vi "UHR-Fleezers Control (host) - 12.7b.vi"() -> ()   [LabVIEW 2012] (continued)
    n2530 = Bundle By Name(cluster=w3378, "Set 1"=w3366, "Set 2"=w3365) -> (→"Trap X AI1 (DMA)":T13)
    n2531 = Cluster To Array(cluster=w3387) -> (array=w3384:string[])
    n2532 = Unbundle(w3244) -> (w3245:u32[])  [unwired: 2 out]
    n2533 = Select(t=-1.0, s="Negate Y Axis", f=1.0) -> (s? t:f=w3328:dbl)
    n2534 = for "Trap Position" {
      tunnel: w3392 -> [w3763] mode=indexing
      tunnel: "Trap Pos. Disp. Downsample" -> [w3762]
      tunnel: w3309 -> [w3760]
      tunnel: w3388 -> [w3759]
      tunnel: w3384 -> [w3757] mode=indexing
      tunnel: [w3756] -> w3298 mode=indexing
      tunnel: w3343 -> [w3754] mode=indexing
      tunnel: w3342 -> [w3752]
      tunnel: w3328 -> [w3751]
      n2535 = call "downsample 1D array - double.vi"("Ave N"=w3762, "Array In"=w3763) -> ("Array Out"=w3761:dbl[])  [unwired: 1 out]
      n2536 = Subtract(x=w3761, y=w3754) -> (x-y=w3755:dbl[])
      n2537 = Multiply(x=w3752, y=w3755) -> (x*y=w3753:dbl[])
      n2538 = Multiply(x=w3751, y=w3753) -> (x*y=w3750:dbl[])
      n2539 = Bundle By Name("Y"=w3750, "dt"=w3760, "t0"=w3759) -> (w3758:waveform(dbl))  [unwired: 1 out]
      n2540 = Set Waveform Attribute(5:w3757, 6:"NI_ChannelName" ("name"), 7:w3758) -> (3:w3756:waveform(dbl))  [unwired: 1 in, 2 out]
    }
    n2541 = To Double Precision Float(number=w3245) -> (double precision float=w3451:dbl[])
    n2542 = local read "Display Period (s)"() -> (w3440:dbl)
    n2543 = Increment(x=w3533) -> (x+1=w3534:dbl)
    n2544 = Index Array(array=w3298, index=0) -> (element=w3302:waveform(dbl))
    n2545 = Index Array(array=w3298, index=1) -> (element=w3297:waveform(dbl))
    n2546 = feedback #7(w3534) -> (w3537:dbl)
    n2547 = Select(t=0, s=w3524, f=w3537) -> (s? t:f=w3530:dbl)
    n2548 = Array Size(array=w3451) -> (size(s)=w3536:i32)
    n2549 = Build Array (concatenate)(w3419, w3555) -> (w3421:waveform(dbl)[])
    "All Signals" <- w3421
    n2550 = Add(x=w3536, y=w3530) -> (x+y=w3531:dbl)
    n2551 = Unbundle By Name(w3302) -> ("Y"=w3303:dbl[])
    n2552 = Divide(x="Bead Sep. Int. Time (s)", y=w3440) -> (x/y=w3338:dbl)
    n2553 = Add(x=w3303, y="FB Trap Pos Offset") -> (x+y=w3301:dbl[])
    "T1 x pos data" <- w3301
    n2554 = Greater?(x=w3531, y=w3533) -> (0:w3532:bool)
    n2555 = feedback #8(w3301) -> (w3340:dbl[])
    n2556 = Build Array (concatenate)(w3301, w3340) -> (w3339:dbl[])
    n2557 = Bundle By Name(cluster=w3302, "Y"=w3301) -> (w3300:waveform(dbl))
    n2558 = Select(t=w3530, s=w3532, f=w3531) -> (s? t:f=w3529:dbl)
    n2559 = feedback-in #7(w3529) -> ()
    n2560 = local read "MCL Scanning"() -> (w3527:bool)
    n2561 = Bundle(w3300, w3297) -> (w3296:cluster{waveform(dbl), waveform(dbl)})  [unwired: 1 out]
    n2562 = Split 1D Array(array=w3339, index=w3338) -> (first subarray=w3332:dbl[])  [unwired: 1 out]
    n2563 = feedback-in #8(w3332) -> ()
    n2564 = Not(x=w3532) -> (.not. x?=w3526:bool)
    n2565 = Cluster To Array(cluster=w3296) -> (array=w3272:waveform(dbl)[])
    "Trap Positions" <- w3272
    n2566 = call-poly <vilib>:"Mean.vi"("X"=w3332) -> ("mean"=w3331:dbl)  [unwired: 1 out]
    "Mean T1 Position (nm)" <- w3331
    n2567 = Subtract(x=w3332, y=w3331) -> (x-y=w3337:dbl[])
    n2568 = Square(x=w3337) -> (x^2=w3336:dbl[])
    n2569 = And(x=w3526, y=w3527) -> (x .and. y?=w3528:bool)
    n2570 = call-poly <vilib>:"Mean.vi"("X"=w3336) -> ("mean"=w3335:dbl)  [unwired: 1 out]
    n2571 = Square Root(x=w3335) -> (sqrt(x)=w3334:dbl)
    n2572 = Or(x=w3528, y=w3524) -> (x .or. y?=w3525:bool)
    n2573 = Equal?(x="Tab Control 6", y=T35."High Res Display") -> (x = y?=w3457:bool)
    n2574 = Multiply(x=10.0, y=w3334) -> (x*y=→"Trap 1 Position RMS (A)":dbl)
    n2575 = case "For displaying the high resolution display (no downsampling)" shown="True" w3457 {
      tunnel: w3423 -> [_ w3783]
      frame False {
      }
      frame True {
        n2576 = Index Array(array=w3783, index="High Res. Display") -> (element=w3784:waveform(dbl))
        n2577 = call <vilib>:"Std Deviation and Variance.vi"("X"=w3784) -> ("mean"=w3791:dbl, "standard deviation"=w3796:dbl)  [unwired: 1 in, 1 out]
        "Mean Intensity" <- w3791
        "Sigma" <- w3796
        n2578 = Subtract(x=w3784, y=w3791) -> (x-y=w3790:waveform(dbl))
        n2579 = Select(t=w3790, s="Subtract mean", f=w3784) -> (s? t:f=→"1 Channel":waveform(dbl))
        n2580 = Divide(x=w3796, y=w3791) -> (x/y=→"Sigma/Mean":dbl)
        n2581 = feedback #9(1) -> (w3785:i32)
        n2582 = Greater Or Equal?(x=w3785, y="Slow mean N ave.") -> (x >= y?=w3798:bool)
        n2583 = Increment(x=w3785) -> (x+1=w3800:i32)
        n2584 = Select(t=1, s=w3798, f=w3800) -> (s? t:f=w3787:i32)
        n2585 = feedback-in #9(w3787) -> ()
        n2586 = feedback #10() -> (w3788:waveform(dbl))  [unwired: 1 out]
        n2587 = case shown="Default" w3785 {
          tunnel: [w3803 w3806] -> w3789
          tunnel: w3788 -> [w3805 _]
          tunnel: w3784 -> [w3804 w3806]
          frame Default {
            n2588 = call-poly <vilib>:"Append Waveforms.vi"("waveform B"=w3804, "waveform A"=w3805) -> ("waveform out"=w3803:waveform(dbl))  [unwired: 1 in, 8 out]
          }
          frame 1 {
          }
        }
        n2589 = feedback-in #10(w3789) -> ()
        n2590 = case shown="True" w3798 {
          tunnel: w3789 -> [_ w3802]
          frame False {
          }
          frame True {
            n2591 = call-poly <vilib>:"Mean.vi"("X"=w3802) -> ("mean"=→"Slow mean":dbl)  [unwired: 1 out]
          }
        }
      }
    }
    n2592 = case "For plotting results of scanning MCL (fluorescence and detection laser images)" shown="True" w3525 {
      tunnel: w3524 -> [_ w3910]
      tunnel: w3533 -> [_ _]
      tunnel: w3423 -> [_ w4039]
      tunnel: w3401 -> [_ w3947]
      tunnel: w3244 -> [_ w3917]
      frame False {
      }
      frame True {
        w3927 = u32 0 items=["Horizontal", "Vertical", "Central", "1st Diagonal", "2nd Diagonal"] ("Type of Symmetry")
        w3954 = u32 0 items=["Horizontal", "Vertical", "Central", "1st Diagonal", "2nd Diagonal"] ("Type of Symmetry")
        w3978 = u32 0 items=["Horizontal", "Vertical", "Central", "1st Diagonal", "2nd Diagonal"] ("Type of Symmetry")
        w3981 = u32 0 items=["Horizontal", "Vertical", "Central", "1st Diagonal", "2nd Diagonal"] ("Type of Symmetry")
        w4010 = u32 0 items=["Horizontal", "Vertical", "Central", "1st Diagonal", "2nd Diagonal"] ("Type of Symmetry")
        n2593 = Unbundle(w3917) -> (w3916:u32[], w3914:u32[], w3912:u32[])
        n2594 = To Double Precision Float(number=w3916) -> (double precision float=w3915:dbl[])
        n2595 = To Double Precision Float(number=w3914) -> (double precision float=w3913:dbl[])
        n2596 = To Double Precision Float(number=w3912) -> (double precision float=w3911:dbl[])
        n2597 = Index Array(array=w4039, index=10) -> (element=w4045:waveform(dbl))
        n2598 = Index Array(array=w4039, index=11) -> (element=w4042:waveform(dbl))
        n2599 = local read "Cycles/step (MCL)"() -> (w3995:u64)
        n2600 = Index Array(array=w4039, index="Channel") -> (element=w4041:waveform(dbl))
        n2601 = Unbundle(w3947) -> ("New Image"=w3946:T2, "New Image"=w3945:T2, "New Image"=w3918:T2, "New Image"=w3919:T2, "New Image"=w3920:T2)
        n2602 = local read "Scan steps (MCL)"() -> (w3906:u64)
        n2603 = Unbundle By Name(w4045) -> ("Y"=w3997:dbl[])
        n2604 = Unbundle By Name(w4042) -> ("Y"=w3999:dbl[])
        n2605 = local read "Scan lines (y)"() -> (w3907:u64)
        n2606 = local read "N APD Samp/step"() -> (w3909:dbl)
        n2607 = Unbundle By Name(w4041) -> ("Y"=w4004:dbl[])
        n2608 = call "downsample 1D array - double.vi"("Ave N"=w3995, "Array In"=w3997) -> ("Array Out"=w3996:dbl[])  [unwired: 1 out]
        n2609 = call "downsample 1D array - double.vi"("Ave N"=w3995, "Array In"=w3999) -> ("Array Out"=w3998:dbl[])  [unwired: 1 out]
        n2610 = call "downsample 1D array - double.vi"("Ave N"=w3995, "Array In"=w4004) -> ("Array Out"=w4003:dbl[])  [unwired: 1 out]
        n2611 = Multiply(x=w3906, y=u64 2) -> (x*y=w3908:u64)
        n2612 = feedback #11(w3913) -> (w3972:dbl[])
        n2613 = Build Array (concatenate)(w3972, w3913) -> (w3971:dbl[])
        n2614 = feedback #12(w3911) -> (w3944:dbl[])
        n2615 = Build Array (concatenate)(w3944, w3911) -> (w3905:dbl[])
        n2616 = Select(t=w3913, s=w3910, f=w3971) -> (s? t:f=w3956:dbl[])
        n2617 = feedback-in #11(w3956) -> ()
        n2618 = Select(t=w3911, s=w3910, f=w3905) -> (s? t:f=w3929:dbl[])
        n2619 = feedback-in #12(w3929) -> ()
        n2620 = feedback #13(w3915) -> (w4065:dbl[])
        n2621 = Build Array (concatenate)(w4065, w3915) -> (w4047:dbl[])
        n2622 = Select(t=w3915, s=w3910, f=w4047) -> (s? t:f=w4051:dbl[])
        n2623 = feedback-in #13(w4051) -> ()
        n2624 = feedback #14(w3996) -> (w4053:dbl[])
        n2625 = Build Array (concatenate)(w4053, w3996) -> (w4044:dbl[])
        n2626 = feedback #15(w4003) -> (w4063:dbl[])
        n2627 = Build Array (concatenate)(w4063, w4003) -> (w4062:dbl[])
        n2628 = feedback #16(w3998) -> (w4055:dbl[])
        n2629 = Build Array (concatenate)(w4055, w3998) -> (w4056:dbl[])
        n2630 = Select(t=w3996, s=w3910, f=w4044) -> (s? t:f=w4000:dbl[])
        n2631 = feedback-in #14(w4000) -> ()
        n2632 = Select(t=w4003, s=w3910, f=w4062) -> (s? t:f=w4002:dbl[])
        n2633 = feedback-in #15(w4002) -> ()
        n2634 = Select(t=w3998, s=w3910, f=w4056) -> (s? t:f=w4001:dbl[])
        n2635 = feedback-in #16(w4001) -> ()
        n2636 = call "integrate 1D array interval - double.vi"("Ave N"=w3909, "Array In"=w3956) -> ("Array Out"=w3967:dbl[])  [unwired: 1 out]
        n2637 = call "integrate 1D array interval - double.vi"("Ave N"=w3909, "Array In"=w3929) -> ("Array Out"=w3940:dbl[])  [unwired: 1 out]
        n2638 = call "integrate 1D array interval - double.vi"("Ave N"=w3909, "Array In"=w4051) -> ("Array Out"=w4050:dbl[])  [unwired: 1 out]
        n2639 = Array Size(array=w3967) -> (size(s)=w3968:i32)
        n2640 = Array Size(array=w3940) -> (size(s)=w3941:i32)
        n2641 = Array Size(array=w4050) -> (size(s)=w4052:i32)
        n2642 = Multiply(x=w3907, y=w3908) -> (x*y=w3970:u64)
        n2643 = Multiply(x=w3907, y=w3908) -> (x*y=w3943:u64)
        n2644 = Multiply(x=w3907, y=w3908) -> (x*y=w4060:u64)
        n2645 = Subtract(x=w3970, y=w3968) -> (x-y=w3961:u64)
        n2646 = call-poly <vilib>:"Mean.vi"("X"=w3967) -> ("mean"=w3958:dbl)  [unwired: 1 out]
        n2647 = Subtract(x=w3943, y=w3941) -> (x-y=w3934:u64)
        n2648 = call-poly <vilib>:"Mean.vi"("X"=w3940) -> ("mean"=w3931:dbl)  [unwired: 1 out]
        n2649 = Subtract(x=w4060, y=w4052) -> (x-y=w3994:u64)
        n2650 = call-poly <vilib>:"Mean.vi"("X"=w4050) -> ("mean"=w3991:dbl)  [unwired: 1 out]
        n2651 = call-poly <vilib>:"Mean.vi"("X"=w4000) -> ("mean"=w3984:dbl)  [unwired: 1 out]
        n2652 = call-poly <vilib>:"Mean.vi"("X"=w4002) -> ("mean"=w3989:dbl)  [unwired: 1 out]
        n2653 = call-poly <vilib>:"Mean.vi"("X"=w4001) -> ("mean"=w3987:dbl)  [unwired: 1 out]
        n2654 = Initialize Array(1.0 ("element"), w3961) -> (w3957:dbl[])
        n2655 = Initialize Array(1.0 ("element"), w3934) -> (w3930:dbl[])
        n2656 = Initialize Array(1.0 ("element"), w3994) -> (w3985:dbl[])
        n2657 = Multiply(x=w3957, y=w3958) -> (x*y=w3959:dbl[])
        n2658 = Multiply(x=w3930, y=w3931) -> (x*y=w3932:dbl[])
        n2659 = Multiply(x=w3985, y=w3991) -> (x*y=w3992:dbl[])
        n2660 = Multiply(x=w3985, y=w3987) -> (x*y=w3988:dbl[])
        n2661 = Multiply(x=w3985, y=w3989) -> (x*y=w3990:dbl[])
        n2662 = Multiply(x=w3985, y=w3984) -> (x*y=w3986:dbl[])
        n2663 = Build Array (concatenate)(w3967, w3959) -> (w3969:dbl[])
        n2664 = Build Array (concatenate)(w3940, w3932) -> (w3942:dbl[])
        n2665 = Build Array (concatenate)(w4050, w3992) -> (w4059:dbl[])
        n2666 = Build Array (concatenate)(w4000, w3986) -> (w4054:dbl[])
        n2667 = Build Array (concatenate)(w4002, w3990) -> (w4058:dbl[])
        n2668 = Build Array (concatenate)(w4001, w3988) -> (w4057:dbl[])
        n2669 = Reshape Array(w3969, w3907, w3908) -> (w3965:dbl[][])
        n2670 = Reshape Array(w3942, w3907, w3908) -> (w3938:dbl[][])
        n2671 = Reshape Array(w4059, w3907, w3908) -> (w4037:dbl[][])
        n2672 = Reshape Array(w4054, w3907, w3908) -> (w4020:dbl[][])
        n2673 = Reshape Array(w4058, w3907, w3908) -> (w4012:dbl[][])
        n2674 = Reshape Array(w4057, w3907, w3908) -> (w4027:dbl[][])
        n2675 = Array Subset(array=w3965, index (col)=0 ("index"), length (col)=w3906) -> (w3964:dbl[][])  [unwired: 2 in]
        n2676 = Array Subset(array=w3965, index (col)=w3906) -> (w3962:dbl[][])  [unwired: 3 in]
        n2677 = Array Subset(array=w3938, index (col)=0 ("index"), length (col)=w3906) -> (w3937:dbl[][])  [unwired: 2 in]
        n2678 = Array Subset(array=w3938, index (col)=w3906) -> (w3935:dbl[][])  [unwired: 3 in]
        n2679 = Array Subset(array=w4027, index (col)=0 ("index"), length (col)=w3906) -> (w4032:dbl[][])  [unwired: 2 in]
        n2680 = Array Subset(array=w4027, index (col)=w3906) -> (w4030:dbl[][])  [unwired: 3 in]
        n2681 = Array Subset(array=w4037, index (col)=0 ("index"), length (col)=w3906) -> (w4036:dbl[][])  [unwired: 2 in]
        n2682 = Array Subset(array=w4037, index (col)=w3906) -> (w4034:dbl[][])  [unwired: 3 in]
        n2683 = Array Subset(array=w4012, index (col)=0 ("index"), length (col)=w3906) -> (w4018:dbl[][])  [unwired: 2 in]
        n2684 = Array Subset(array=w4012, index (col)=w3906) -> (w4016:dbl[][])  [unwired: 3 in]
        n2685 = Array Subset(array=w4020, index (col)=0 ("index"), length (col)=w3906) -> (w4025:dbl[][])  [unwired: 2 in]
        n2686 = Array Subset(array=w4020, index (col)=w3906) -> (w4023:dbl[][])  [unwired: 3 in]
        n2687 = for {
          tunnel: w3964 -> [w4069] mode=indexing
          tunnel: [w4068] -> w3963 mode=indexing
          workers-P: _ -> [_]
          n2688 = Reverse 1D Array(array=w4069) -> (reversed array=w4068:dbl[])
        }
        n2689 = for {
          tunnel: w3937 -> [w4067] mode=indexing
          tunnel: [w4066] -> w3936 mode=indexing
          workers-P: _ -> [_]
          n2690 = Reverse 1D Array(array=w4067) -> (reversed array=w4066:dbl[])
        }
        n2691 = for {
          tunnel: w4032 -> [w4075] mode=indexing
          tunnel: [w4074] -> w4031 mode=indexing
          workers-P: _ -> [_]
          n2692 = Reverse 1D Array(array=w4075) -> (reversed array=w4074:dbl[])
        }
        n2693 = for {
          tunnel: w4036 -> [w4077] mode=indexing
          tunnel: [w4076] -> w4035 mode=indexing
          workers-P: _ -> [_]
          n2694 = Reverse 1D Array(array=w4077) -> (reversed array=w4076:dbl[])
        }
        n2695 = for {
          tunnel: w4018 -> [w4071] mode=indexing
          tunnel: [w4070] -> w4017 mode=indexing
          workers-P: _ -> [_]
          n2696 = Reverse 1D Array(array=w4071) -> (reversed array=w4070:dbl[])
        }
        n2697 = for {
          tunnel: w4025 -> [w4073] mode=indexing
          tunnel: [w4072] -> w4024 mode=indexing
          workers-P: _ -> [_]
          n2698 = Reverse 1D Array(array=w4073) -> (reversed array=w4072:dbl[])
        }
        n2699 = Index Array(array=w4037, index (row)=0) -> (element=→"Waveform Graph":dbl[])  [unwired: 1 in]
        n2700 = Add(x=w3963, y=w3962) -> (x+y=w3949:dbl[][])
        n2701 = Add(x=w3936, y=w3935) -> (x+y=w3922:dbl[][])
        n2702 = Add(x=w4031, y=w4030) -> (x+y=w4029:dbl[][])
        n2703 = Add(x=w4035, y=w4034) -> (x+y=w4009:dbl[][])
        n2704 = Add(x=w4017, y=w4016) -> (x+y=w4015:dbl[][])
        n2705 = Add(x=w4024, y=w4023) -> (x+y=w4022:dbl[][])
        n2706 = Divide(x=w4015, y=2) -> (x/y=w4013:dbl[][])
        n2707 = Divide(x=w4029, y=2) -> (x/y=w3974:dbl[][])
        n2708 = To Single Precision Float(number=w4009) -> (single precision float=w4008:sgl[][])
        n2709 = To Single Precision Float(number=w3949) -> (single precision float=w3953:sgl[][])
        n2710 = To Single Precision Float(number=w3922) -> (single precision float=w3926:sgl[][])
        n2711 = Divide(x=w4022, y=2) -> (x/y=w3976:dbl[][])
        n2712 = Transpose 2D Array(2D array=w4013) -> (transposed array=→"Data map":dbl[][])
        n2713 = To Single Precision Float(number=w3974) -> (single precision float=w3980:sgl[][])
        n2714 = To Single Precision Float(number=w3976) -> (single precision float=w3977:sgl[][])
        n2715 = call "IMAQ ArrayToImage"("Image Pixels (Float)"=w4008, "Image"=w3946) -> ("Image Out"=w4011:T2)  [unwired: 8 in, 1 out]
        n2716 = call "IMAQ ArrayToImage"("Image Pixels (Float)"=w3953, "Image"=w3945) -> ("Image Out"=w3955:T2)  [unwired: 8 in, 1 out]
        n2717 = call "IMAQ ArrayToImage"("Image Pixels (Float)"=w3926, "Image"=w3918) -> ("Image Out"=w3928:T2)  [unwired: 8 in, 1 out]
        n2718 = call "IMAQ ArrayToImage"("Image Pixels (Float)"=w3980, "Image"=w3919) -> ("Image Out"=w3982:T2)  [unwired: 8 in, 1 out]
        n2719 = call "IMAQ Symmetry"("Type of Symmetry"=w4010, "Image Src"=w4011) -> ("Image Dst Out"=w4006:T2)  [unwired: 3 in, 1 out]
        n2720 = call "IMAQ ArrayToImage"("Image Pixels (Float)"=w3977, "Image"=w3920) -> ("Image Out"=w3979:T2)  [unwired: 8 in, 1 out]
        n2721 = call "IMAQ Symmetry"("Type of Symmetry"=w3954, "Image Src"=w3955) -> ("Image Dst Out"=w3951:T2)  [unwired: 3 in, 1 out]
        n2722 = call "IMAQ Symmetry"("Type of Symmetry"=w3927, "Image Src"=w3928) -> ("Image Dst Out"=w3924:T2)  [unwired: 3 in, 1 out]
        n2723 = call "IMAQ Symmetry"("Type of Symmetry"=w3981, "Image Src"=w3982) -> ("Image Dst Out"=→"Detection Laser X":T2)  [unwired: 3 in, 1 out]
        n2724 = call "IMAQ Symmetry"("Type of Symmetry"=w3978, "Image Src"=w3979) -> ("Image Dst Out"=→"Detection Laser Y":T2)  [unwired: 3 in, 1 out]
        n2725 = call "IMAQ Set Simple Calibration"("Calibration Axis Info"=T36 {"Origin Pixel"={"X"=0.0, "Y"=0.0}, "Angle Relative to Horizontal (deg)"=0.0, "Axis Reference"=0}, "Grid Descriptor"=T37 {"X Step"=0.3, "Y Step"=0.3, "Unit"=enum."Undefined"}, "Image"=w4006) -> ("Calibrated Image"=→"APD 1":T2)  [unwired: 7 in, 1 out]
        n2726 = call "IMAQ Set Simple Calibration"("Calibration Axis Info"=T36 {"Origin Pixel"={"X"=0.0, "Y"=0.0}, "Angle Relative to Horizontal (deg)"=0.0, "Axis Reference"=0}, "Grid Descriptor"=T37 {"X Step"=0.3, "Y Step"=0.3, "Unit"=enum."Undefined"}, "Image"=w3951) -> ("Calibrated Image"=→"APD 2":T2)  [unwired: 7 in, 1 out]
        n2727 = call "IMAQ Set Simple Calibration"("Calibration Axis Info"=T36 {"Origin Pixel"={"X"=0.0, "Y"=0.0}, "Angle Relative to Horizontal (deg)"=0.0, "Axis Reference"=0}, "Grid Descriptor"=T37 {"X Step"=0.3, "Y Step"=0.3, "Unit"=enum."Undefined"}, "Image"=w3924) -> ("Calibrated Image"=→"APD 3":T2)  [unwired: 7 in, 1 out]
      }
    }
    n2728 = case "For computing FFTs for display" shown="True" "Compute FFT" {
      tunnel: w3423 -> [_ w4549]
      frame False {
      }
      frame True {
        n2729 = Build Array("FFT 1 Choice 1", "FFT 1 Choice 2", "FFT 2 Choice 1", "FFT 2 Choice 2") -> (w4542:u16[])
        n2730 = Array Size(array=w4549) -> (size(s)=w4548:i32)
        n2731 = feedback-in #17(w4542) -> ()
        n2732 = feedback #17(u16[] [100, 100, 100, 100]) -> (w4543:u16[])
        n2733 = feedback-in #18("# Spectra to Ave.") -> ()
        n2734 = feedback #18("# Spectra to Ave.") -> (w4540:dbl)
        n2735 = Not Equal?(x="# Spectra to Ave.", y=w4540) -> (x != y?=w4539:bool)
        n2736 = Not Equal?(x=w4542, y=w4543) -> (x != y?=w4541:bool)
        n2737 = feedback #19(1.0) -> (w4526:dbl)
        n2738 = Compound Arithmetic op=OR("Reset FFT", w4541, w4539) -> (w4524:bool)
        n2739 = Select(t=1.0, s=w4524, f=w4526) -> (s? t:f=w4528:dbl)
        n2740 = Greater?(x=w4528, y="# Spectra to Ave.") -> (0:w4547:bool)
        n2741 = Increment(x=w4528) -> (x+1=w4527:dbl)
        n2742 = feedback-in #19(w4527) -> ()
        n2743 = local read "DMA Update Period (s)"() -> (w4522:dbl)
        n2744 = Multiply(x="# Spectra to Ave.", y=w4522) -> (x*y=→"Ave. Time (s)":dbl)
        n2745 = Build Array(cluster{"f0":dbl, "df":dbl, "magnitude":dbl[]} {"f0"=0.0, "df"=0.0, "magnitude"=[]} ("PSD")) -> (w4531:cluster{"f0":dbl, "df":dbl, "magnitude":dbl[]}[])
        n2746 = Build Array(w4531, w4531, w4531, w4531) -> (w4533:T46)
        n2747 = feedback #20(w4533) -> (w4538:T46)
        n2748 = for {
          N: 4 -> [_]
          tunnel: w4542 -> [w4571] mode=indexing
          tunnel: w4549 -> [w4572]
          tunnel: w4548 -> [w4574]
          tunnel: w4524 -> [w4567]
          tunnel: w4547 -> [w4566]
          tunnel: "# Spectra to Ave." -> [w4565]
          tunnel: [w4564] -> w4537 mode=indexing
          tunnel: w4538 -> [w4569] mode=indexing
          tunnel: [w4568] -> w4525 mode=indexing
          tunnel: w4528 -> [w4563]
          n2749 = Less?(x=w4571, y=w4574) -> (x < y?=w4573:bool)
          n2750 = Index Array(array=w4572, index=w4571) -> (element=w4570:waveform(dbl))
          n2751 = case shown="True" w4573 {
            tunnel: w4570 -> [_ w4591]
            tunnel: w4569 -> [w4576 w4589]
            tunnel: [w4576 w4577] -> w4568
            tunnel: w4567 -> [_ w4588]
            tunnel: w4566 -> [_ w4581]
            tunnel: w4565 -> [_ w4580]
            tunnel: [cluster{"f0":dbl, "df":dbl, "magnitude":dbl[]} {"f0"=0.0, "df"=0.0, "magnitude"=[]} ("PSD") w4582] -> w4564
            tunnel: w4563 -> [_ w4579]
            frame False {
            }
            frame True {
              n2752 = call <vilib>:"Std Deviation and Variance.vi"("X"=w4591) -> ("mean"=w4592:dbl)  [unwired: 1 in, 2 out]
              n2753 = Subtract(x=w4591, y=w4592) -> (x-y=w4590:waveform(dbl))
              n2754 = xnode "Spectral Measurements"("Signals"=w4590) -> ("PSD"=w4584:cluster{"f0":dbl, "df":dbl, "magnitude":dbl[]})  [unwired: 1 in, 1 out]
              n2755 = case shown="False" w4588 {
                tunnel: w4589 -> [w4601 _]
                tunnel: [w4597 w4606] -> w4577
                tunnel: w4584 -> [w4600 w4607]
                tunnel: w4581 -> [w4599 _]
                frame False {
                  n2756 = Build Array (concatenate)(w4601, w4600) -> (w4598:cluster{"f0":dbl, "df":dbl, "magnitude":dbl[]}[])
                  n2757 = case shown="True" w4599 {
                    tunnel: w4598 -> [w4602 w4605]
                    tunnel: [w4602 w4603] -> w4597
                    frame False {
                    }
                    frame True {
                      n2758 = Delete From Array(array=w4605, index=0) -> (array with subset deleted=w4603:cluster{"f0":dbl, "df":dbl, "magnitude":dbl[]}[])  [unwired: 1 in, 1 out]
                    }
                  }
                }
                frame True {
                  n2759 = Build Array(w4607) -> (w4606:cluster{"f0":dbl, "df":dbl, "magnitude":dbl[]}[])
                }
              }
              n2760 = for {
                tunnel: w4577 -> [w4596] mode=indexing
                tunnel: [w4595] -> w4587 mode=indexing
                workers-P: _ -> [_]
                n2761 = Unbundle By Name(w4596) -> ("magnitude"=w4595:dbl[])
              }
              n2762 = Transpose 2D Array(2D array=w4587) -> (transposed array=w4586:dbl[][])
              n2763 = for {
                tunnel: w4586 -> [w4594] mode=indexing
                tunnel: [w4593] -> w4585 mode=indexing
                workers-P: _ -> [_]
                n2764 = Add Array Elements(numeric array=w4594) -> (sum=w4593:dbl)
              }
              n2765 = Select(t=w4580, s=w4581, f=w4579) -> (s? t:f=w4578:dbl)
              n2766 = Divide(x=w4585, y=w4578) -> (x/y=w4583:dbl[])
              n2767 = Bundle By Name(cluster=w4584, "magnitude"=w4583) -> (w4582:cluster{"f0":dbl, "df":dbl, "magnitude":dbl[]})
            }
          }
        }
        n2768 = case shown="True" w4524 {
          tunnel: w4525 -> [w4556 w4562]
          tunnel: [w4556 w4557] -> w4523
          frame False {
          }
          frame True {
            n2769 = Array Subset(array=w4562, index (row)=0 ("index"), length (row)=4 ("length"), index (col)=0 ("index"), length (col)=1 ("length")) -> (w4557:T46)
          }
        }
        n2770 = feedback-in #20(w4523) -> ()
        n2771 = Split 1D Array(array=w4537, index=2) -> (first subarray=→"FFT 1":cluster{"f0":dbl, "df":dbl, "magnitude":dbl[]}[], second subarray=→"FFT 2":cluster{"f0":dbl, "df":dbl, "magnitude":dbl[]}[])
      }
    }
    n2772 = Index Array(array=w3421, index=4) -> (element=w3477:waveform(dbl))
    n2773 = Index Array(array=w3421, index=7) -> (element=w3474:waveform(dbl))
    n2774 = Divide(x="T1 offset_x (mV)", y=1000.0) -> (x/y=w3478:dbl)
    n2775 = feedback-in #21("Calibration") -> ()
    n2776 = feedback #21(u16 1 ("Calibration")) -> (w3496:u16)
    n2777 = Divide(x="T2 offset_x (mV)", y=1000.0) -> (x/y=w3476:dbl)
    n2778 = case shown="2" "Calibration" {
      tunnel: "T1 alpha_x (nm/V)" -> [_ w3870 w3891]
      tunnel: "T1 kappa_x (pN/nm)" -> [_ _ w3881]
      tunnel: "T2 alpha_x (nm/V)" -> [_ w3869 w3889]
      tunnel: "T2 kappa_x (pN/nm)" -> [_ _ w3882]
      tunnel: w3477 -> [w3852 w3867 w3887]
      tunnel: w3474 -> [w3851 w3865 w3885]
      tunnel: [w3852 w3864 w3884] -> w3505
      tunnel: [w3851 w3863 w3883] -> w3504
      tunnel: ["T1 X (V)" ("Label.Text") "T1 X (nm)" ("Label.Text") "T1 X (pN)" ("Label.Text")] -> w3493
      tunnel: ["T2 X (V)" ("Label.Text") "T2 X (nm)" ("Label.Text") "T2 X (pN)" ("Label.Text")] -> w3492
      tunnel: ["Position (V)" ("Label.Text") "Position (nm)" ("Label.Text") "Force (pN)" ("Label.Text")] -> w3494
      tunnel: w3476 -> [_ w3855 w3874]
      tunnel: w3478 -> [_ w3858 w3876]
      tunnel: ["Mean (V)" ("Label.Text") "Mean (nm)" ("Label.Text") "Mean (pN)" ("Label.Text")] -> w3489
      tunnel: ["Difference (V)" ("Label.Text") "Difference (nm)" ("Label.Text") "Difference (pN)" ("Label.Text")] -> w3429
      frame 0, Default {
      }
      frame 1 {
        n2779 = Unbundle By Name(w3867) -> ("Y"=w3871:dbl[])
        n2780 = Unbundle By Name(w3865) -> ("Y"=w3856:dbl[])
        n2781 = Subtract(x=w3871, y=w3858) -> (x-y=w3859:dbl[])
        n2782 = Subtract(x=w3856, y=w3855) -> (x-y=w3857:dbl[])
        n2783 = Multiply(x=w3857, y=w3869) -> (x*y=w3866:dbl[])
        n2784 = Multiply(x=w3870, y=w3859) -> (x*y=w3868:dbl[])
        n2785 = Bundle By Name(cluster=w3865, "Y"=w3866) -> (w3863:waveform(dbl))
        n2786 = Bundle By Name(cluster=w3867, "Y"=w3868) -> (w3864:waveform(dbl))
      }
      frame 2 {
        n2787 = Unbundle By Name(w3887) -> ("Y"=w3892:dbl[])
        n2788 = Unbundle By Name(w3885) -> ("Y"=w3890:dbl[])
        n2789 = Subtract(x=w3890, y=w3874) -> (x-y=w3875:dbl[])
        n2790 = Subtract(x=w3892, y=w3876) -> (x-y=w3877:dbl[])
        n2791 = Compound Arithmetic op=MULTIPLY(w3875, w3889, w3882) -> (w3886:dbl[])
        n2792 = Compound Arithmetic op=MULTIPLY(w3881, w3891, w3877) -> (w3888:dbl[])
        n2793 = Bundle By Name(cluster=w3885, "Y"=w3886) -> (w3883:waveform(dbl))
        n2794 = Bundle By Name(cluster=w3887, "Y"=w3888) -> (w3884:waveform(dbl))
      }
    }
    n2795 = case shown="True" "Read Lateness and Rel Phase" {
      tunnel: w3295 -> [w3807 w3840]
      tunnel: w3294 -> [w3808 w3839]
      tunnel: [w3807 w3812] -> w3471
      tunnel: [w3808 w3811] -> w3470
      frame False {
      }
      frame True {
        n2796 = xnode "Read/Write Control"("FPGA VI Reference In"=w3840, "error in"=w3839) -> ("FPGA VI Reference Out"=w3814:T20, "error out"=w3813:errorcluster, "GI Relative phase"=→"GI relative phase":i16, "Relative phase"=→"Relative phase (AI1)":i16, "AI Late Counter"=→"Late Counter (AI1)":u8, "GI Late Counter"=→"GI Late Counter":u8, "MCL Late Counter"=→"MCL Late Counter":u8, "MCL Relative Phase"=→"Relative Phase (MCL)":i16, "APD Acq Relative Phase"=→"APD Acq Relative Phase":i16, "APD 1 Gate Relative Phase"=→"APD 1 Gate Relative Phase":i16, "APD 2 Gate Relative Phase"=→"APD 2 Gate Relative Phase":i16, "APD Acq Late Counter"=→"APD Acq Late Counter":u8, "APD 1 Gate Late Counter"=→"APD 1 Gate Late Counter":u8, "APD 2 Gate Late Counter"=→"APD 2 Gate Late Counter":u8, "Green FB Relative Phase"=→"Relative phase (Green FB)":i16, "GI Relative phase 2"=→"GI relative phase 2":i16, "GI Late Counter 2"=→"GI Late Counter 2":u8, "Trap Pos FIFO Timeout"=→"Trap Pos FIFO Timeout":u16, "Trap AI FIFO Timeout"=→"Trap AI FIFO Timeout":u16, "RI Late Counter"=→"RI Late Counter":u8, "RI Relative phase"=→"RI relative phase":i16, "Green Late Counter"=→"Green AI Late Counter":u8, "BI Late Counter (AO)"=→"Late Counter (BI AO)":u8, "Blue Late Counter (D)"=→"Late Counter (BI DO)":u8, "BI Relative phase (AO)"=→"Relative phase (BI AO)":i16, "BI Relative phase (D)"=→"Relative phase (BI DO)":i16)
        n2797 = xnode "Read/Write Control"("FPGA VI Reference In"=w3814, "error in"=w3813) -> ("FPGA VI Reference Out"=w3812:T20, "error out"=w3811:errorcluster, "APD 3 Gate Late Counter"=→"APD 3 Gate Late Counter":u8, "APD 3 Gate Relative Phase"=→"APD 3 Gate Relative Phase":i16)
      }
    }
    n2798 = Not Equal?(x=w3496, y="Calibration") -> (x != y?=w3455:bool)
    n2799 = case shown="True" w3455 {
      tunnel: w3494 -> [_ w3845]
      tunnel: w3493 -> [_ w3844]
      tunnel: w3492 -> [_ w3843]
      tunnel: w3489 -> [_ w3842]
      tunnel: w3429 -> [_ w3841]
      frame False {
      }
      frame True {
        n2800 = property on="Force" class="WFChart (strict)"("YScale.NameLbl.Text"=w3845) -> ()  [unwired: 2 in, 2 out]
        n2801 = property on="T2 X" class="DigNum (strict)"("Caption.Text"=w3843) -> ()  [unwired: 2 in, 2 out]
        n2802 = property on="T1 X" class="DigNum (strict)"("Caption.Text"=w3844) -> ()  [unwired: 2 in, 2 out]
        n2803 = property on="Mean" class="DigNum (strict)"("Caption.Text"=w3842) -> ()  [unwired: 2 in, 2 out]
        n2804 = property on="Difference" class="DigNum (strict)"("Caption.Text"=w3841) -> ()  [unwired: 2 in, 2 out]
      }
    }
    n2805 = Unbundle By Name(w3477) -> ("Y"=w3480:dbl[])
    n2806 = Unbundle By Name(w3474) -> ("Y"=w3483:dbl[])
    n2807 = Subtract(x=w3480, y=w3478) -> (x-y=w3481:dbl[])
    n2808 = Subtract(x=w3483, y=w3476) -> (x-y=w3482:dbl[])
    n2809 = Multiply(x=w3482, y="T2 alpha_x (nm/V)") -> (x*y=w3277:dbl[])
    n2810 = Multiply(x="T1 alpha_x (nm/V)", y=w3481) -> (x*y=w3278:dbl[])
    n2811 = Not(x="Trap Trig. Fl.") -> (.not. x?=w3314:bool)
    n2812 = Multiply(x=w3504, y=-1.0) -> (x*y=w3485:waveform(dbl))
    n2813 = Subtract(x=w3278, y=w3277) -> (x-y=w3473:dbl[])
    n2814 = Unbundle By Name(w3504) -> ("Y"=w3445:dbl[])
    n2815 = Unbundle By Name(w3505) -> ("Y"=w3279:dbl[])
    n2816 = Negate(x=w3473) -> (-x=w3275:dbl[])
    n2817 = Build Array(w3505, w3485) -> (→"Force":waveform(dbl)[])
    n2818 = Subtract(x=w3275, y="Offset (nm)") -> (x-y=w3443:dbl[])
    n2819 = call-poly <vilib>:"Mean.vi"("X"=w3445) -> ("mean"=w3281:dbl)  [unwired: 1 out]
    "T2 X" <- w3281
    n2820 = Negate(x=w3445) -> (-x=w3446:dbl[])
    n2821 = call-poly <vilib>:"Mean.vi"("X"=w3279) -> ("mean"=w3282:dbl)  [unwired: 1 out]
    "T1 X" <- w3282
    n2822 = Negate(x=w3281) -> (-x=w3280:dbl)
    n2823 = Bundle By Name(cluster=w3477, "Y"=w3443) -> (w3420:waveform(dbl))
    "Bead Separation" <- w3420
    n2824 = Add(x=w3279, y=w3446) -> (x+y=w3447:dbl[])
    n2825 = Add(x=w3282, y=w3280) -> (x+y=w3491:dbl)
    n2826 = Subtract(x=w3282, y=w3280) -> (x-y=→"Difference":dbl)
    n2827 = Divide(x=w3447, y=2.0) -> (x/y=→"Vec Mean of T1 T2":dbl[])
    n2828 = Divide(x=w3491, y=2.0) -> (x/y=w3449:dbl)
    "Mean" <- w3449
    n2829 = feedback-in #22("Trap Trig. Fl.") -> ()
    n2830 = feedback #22("Trap Trig. Fl.") -> (w3312:bool)
    n2831 = And(x=w3314, y=w3312) -> (x .and. y?=w3313:bool)
    n2832 = case "If have just turned off triggering" shown="True" w3313 {
      tunnel: w3295 -> [_ w3642]
      tunnel: w3294 -> [_ w3641]
      frame False {
      }
      frame True {
        w3640 = FALSE ("FPGA Trap Trig")
        n2833 = xnode "Read/Write Control"("FPGA VI Reference In"=w3642, "error in"=w3641, "FPGA Trap Trig"=w3640) -> ("FPGA VI Reference Out"=w3639:T20, "error out"=w3638:errorcluster)
        n2834 = xnode "Read/Write Control"("FPGA VI Reference In"=w3639, "error in"=w3638, "TTrig?"=w3640) -> ()  [unwired: 2 out]
        n2835 = local write "Initializing"(FALSE ("Initializing")) -> ()
        n2836 = local write "Triggered"(FALSE ("Triggered")) -> ()
        n2837 = local write "Waiting"(FALSE ("Waiting")) -> ()
      }
    }
    n2838 = Not(x=w3312) -> (.not. x?=w3325:bool)
    n2839 = And(x="Trap Trig. Fl.", y=w3325) -> (x .and. y?=w3322:bool)
    n2840 = local read "Tether"() -> (w3450:bool)
    n2841 = Or(x=w3322, y="Reinitialize") -> (x .or. y?=w3308:bool)
    n2842 = feedback #23(w3318) -> (w3323:string)
    n2843 = Select(t=w3318, s=w3322, f=w3323) -> (s? t:f=w3317:string)
    n2844 = Select(t=w3318, s="Reinitialize", f=w3317) -> (s? t:f=w3316:string)
    n2845 = feedback #24(0) -> (w3320:i32)
    n2846 = feedback #25(w3443) -> (w3442:dbl[])
    n2847 = Build Array (concatenate)(w3443, w3442) -> (w3276:dbl[])
    n2848 = case "For determining if there is a tether still" shown="True" w3450 {
      tunnel: w3449 -> [_ w3766]
      frame False {
      }
      frame True {
        n2849 = Greater?(x="Lost Tether Alarm Threshold (pN)", y=w3766) -> (0:w3764:bool)
        n2850 = case shown="True" w3764 {
          frame False {
          }
          frame True {
            w3767 = FALSE ("Value (Signaling)")
            n2851 = flat-sequence {
              frame #0 {
                # "stop only if saving"
                n2852 = local read "Saving..."() -> (w3779:bool)
                n2853 = And(x=w3779, y="TA Cancel Save?") -> (x .and. y?=w3778:bool)
                n2854 = local write "Stop Saving"(w3778) -> ()
              }
              frame #1 {
                n2855 = case shown="True" "TA Green Off?" {
                  frame False {
                  }
                  frame True {
                    w3782 = FALSE ("Fl. Triggered...")
                    n2856 = local write "Fl. Triggered..."(w3782) -> ()
                    n2857 = property on="Green Laser ON" class="Bool (strict)"("Val(Sgnl)"=w3782) -> ()  [unwired: 2 in, 2 out]
                  }
                }
              }
            }
            n2858 = local read "Time tether formed"() -> (w3773:timestamp)
            n2859 = Get Date/Time In Seconds() -> (seconds since 1Jan1904=w3774:timestamp)
            n2860 = Subtract(x=w3774, y=w3773) -> (x-y=w3772:dbl)
            n2861 = Number To Decimal String(number=w3772) -> (decimal integer string=w3769:string)  [unwired: 1 out]
            n2862 = local read "Messages"() -> (w3776:string)
            n2863 = call <vilib>:"Beep.vi"() -> ()  [unwired: 3 in, 9 out]
            n2864 = Concatenate Strings("Lost tether (" ("Message to add"), w3769, " s)." ("string")) -> (w3771:string)
            n2865 = local write "Tether"(FALSE ("Tether")) -> ()
            n2866 = call "Update messages.vi"("Message to add"=w3771, "Old message string"=w3776) -> ("New message string"=w3775:string)
            n2867 = local write "Messages"(w3775) -> ()
            n2868 = property on="Fl. Triggered..." class="Bool (strict)"("Val(Sgnl)"=w3767) -> ()  [unwired: 2 in, 2 out]
            n2869 = local write "Dip for Protein"(w3767) -> ()
            n2870 = property on="Trap Pos. FB ON" class="Bool (strict)"("Val(Sgnl)"=w3767) -> ()  [unwired: 2 in, 2 out]
            n2871 = property on="Trap Trig. Fl." class="Bool (strict)"("Val(Sgnl)"=w3767) -> ()  [unwired: 2 in, 2 out]
          }
        }
      }
    }
    n2872 = case "For triggering actions based on the trap position (e.g., turning the excitation laser on if trap under feedback moves so far)" shown="True" "Trap Trig. Fl." {
      tunnel: w3303 -> [_ w3655]
      tunnel: w3316 -> [_ w3654]
      tunnel: ["" ("t") w3653] -> w3324
      tunnel: w3308 -> [_ w3652]
      tunnel: [0 ("t") w3651] -> w3321
      tunnel: w3320 -> [_ w3650]
      tunnel: w3295 -> [_ w3649]
      tunnel: w3294 -> [_ w3648]
      frame False {
      }
      frame True {
        n2873 = case shown="\"Wait for trigger\"" w3654 {
          tunnel: w3655 -> [w3672 _ _ w3720]
          tunnel: [w3669 w3701 "" ("t") w3723] -> w3653
          tunnel: w3652 -> [_ _ _ w3711]
          tunnel: [w3668 w3698 0 ("t") w3712] -> w3651
          tunnel: w3650 -> [_ w3700 _ w3718]
          tunnel: w3649 -> [w3657 w3695 _ w3714]
          tunnel: w3648 -> [w3656 w3694 _ w3713]
          frame "Wait for trigger" {
            n2874 = local read "Trap Trig. (FPGA)"() -> (w3660:bool)
            n2875 = Subtract(x=w3672, y="Mean T1 Position\nto compare (nm)") -> (x-y=w3665:dbl[])
            n2876 = call <vilib>:"Std Deviation and Variance.vi"("X"=w3665) -> ("mean"=→"mean":dbl, "standard deviation"=→"standard\ndeviation":dbl)  [unwired: 1 in, 1 out]
            n2877 = Array Max & Min(array=w3665) -> (max value=→"max value":dbl, min value=→"min value":dbl)  [unwired: 2 out]
            n2878 = Greater?(x=w3665, y="Threshold (nm)") -> (0:w3675:bool[])
            n2879 = case shown="True" w3660 {
              tunnel: w3657 -> [_ w3681]
              tunnel: w3656 -> [_ w3680]
              tunnel: [FALSE ("TTrig?") w3679] -> w3663
              frame False {
              }
              frame True {
                n2880 = xnode "Read/Write Control"("FPGA VI Reference In"=w3681, "error in"=w3680) -> ("TTrig?"=w3679:bool)  [unwired: 2 out]
              }
            }
            n2881 = Or Array Elements(Boolean array=w3675) -> (logical OR=w3662:bool)
            n2882 = Select(t=w3663, s=w3660, f=w3662) -> (s? t:f=w3661:bool)
            n2883 = Not(x=w3660) -> (.not. x?=w3659:bool)
            n2884 = And(x=w3661, y=w3659) -> (x .and. y?=w3658:bool)
            n2885 = Select(t="Triggered", s=w3661, f="Wait for trigger") -> (s? t:f=w3669:string)
            n2886 = case shown="True" w3661 {
              tunnel: [0 0] -> w3668
              tunnel: w3657 -> [_ w3686]
              tunnel: w3656 -> [_ w3685]
              frame False {
                "Waiting" <- TRUE ("Waiting")
              }
              frame True {
                n2887 = xnode "Read/Write Control"("FPGA VI Reference In"=w3686, "error in"=w3685, "TTrig?"=FALSE) -> ()  [unwired: 2 out]
                n2888 = local read "Messages"() -> (w3689:string)
                n2889 = call <vilib>:"Beep.vi"() -> ()  [unwired: 12 in]
                n2890 = call "Update messages.vi"("Message to add"="Unwinding trigger.", "Old message string"=w3689) -> ("New message string"=w3690:string)
                n2891 = local write "Messages"(w3690) -> ()
                n2892 = local write "Waiting"(FALSE ("Waiting")) -> ()
                "Triggered" <- TRUE ("Triggered")
              }
            }
            n2893 = case "Only need to turn on laser if host triggered" shown="True" w3658 {
              frame False {
              }
              frame True {
                n2894 = property on="Green Laser ON" class="Bool (strict)"("Val(Sgnl)"=TRUE ("Value (Signaling)")) -> ()  [unwired: 2 in, 2 out]
              }
            }
          }
          frame "Triggered" {
            n2895 = local read "Trap Trig. (FPGA)"() -> (w3697:bool)
            n2896 = Increment(x=w3700) -> (x+1=w3698:i32)
            n2897 = Greater Or Equal?(x=w3698, y="Fl. ON time (n)") -> (x >= y?=w3696:bool)
            n2898 = Select(t="Wait for trigger", s=w3696, f="Triggered" ("t")) -> (s? t:f=w3701:string)
            n2899 = And(x=w3696, y=w3697) -> (x .and. y?=w3693:bool)
            n2900 = case shown="True" w3693 {
              tunnel: w3695 -> [_ w3705]
              tunnel: w3694 -> [_ w3704]
              frame False {
              }
              frame True {
                n2901 = xnode "Read/Write Control"("FPGA VI Reference In"=w3705, "error in"=w3704, "FPGA Trap Trig"=TRUE) -> ()  [unwired: 2 out]
              }
            }
            n2902 = case shown="True" w3696 {
              frame False {
              }
              frame True {
                w3707 = FALSE ("Value (Signaling)")
                n2903 = local write "Triggered"(w3707) -> ()
                n2904 = local write "Waiting"(TRUE ("Waiting")) -> ()
                n2905 = property on="Green Laser ON" class="Bool (strict)"("Val(Sgnl)"=w3707) -> ()  [unwired: 2 in, 2 out]
              }
            }
          }
          frame "Do nothing" {
          }
          frame "Initialize", Default {
            n2906 = Increment(x=w3718) -> (x+1=w3722:i32)
            n2907 = Select(t=1, s=w3711, f=w3722) -> (s? t:f=w3712:i32)
            n2908 = feedback #26(w3720) -> (w3726:dbl[])
            n2909 = Build Array (concatenate)(w3720, w3726) -> (w3719:dbl[])
            n2910 = Greater Or Equal?(x=w3712, y="Wait to get offset (n)") -> (x >= y?=w3715:bool)
            n2911 = Select(t=w3720, s=w3711, f=w3719) -> (s? t:f=w3721:dbl[])
            n2912 = feedback-in #26(w3721) -> ()
            n2913 = call-poly <vilib>:"Mean.vi"("X"=w3721) -> ("mean"=w3716:dbl)  [unwired: 1 out]
            n2914 = local write "Mean T1 Position\nto compare (nm)"(w3716) -> ()
            n2915 = case shown="True" w3711 {
              tunnel: w3714 -> [_ w3732]
              tunnel: w3713 -> [_ w3731]
              frame False {
              }
              frame True {
                w3728 = FALSE ("FPGA Trap Trig")
                n2916 = xnode "Read/Write Control"("FPGA VI Reference In"=w3732, "error in"=w3731, "FPGA Trap Trig"=w3728) -> ("FPGA VI Reference Out"=w3730:T20, "error out"=w3729:errorcluster)
                n2917 = xnode "Read/Write Control"("FPGA VI Reference In"=w3730, "error in"=w3729, "TTrig?"=w3728) -> ()  [unwired: 2 out]
              }
            }
            n2918 = Select(t="Wait for trigger", s=w3715, f="Initialize") -> (s? t:f=w3723:string)
            n2919 = case shown="True" w3715 {
              tunnel: w3716 -> [_ w3735]
              tunnel: w3714 -> [_ w3744]
              tunnel: w3713 -> [_ w3743]
              frame False {
                n2920 = local write "Waiting"(FALSE ("Waiting")) -> ()
                "Initializing" <- TRUE ("Initializing")
              }
              frame True {
                n2921 = local read "Threshold (nm)"() -> (w3747:dbl)
                n2922 = local read "AOM X Cal (nm/MHz)"() -> (w3746:dbl)
                n2923 = Add(x=w3735, y=w3747) -> (x+y=w3748:dbl)
                n2924 = Divide(x=w3748, y=w3746) -> (x/y=w3745:dbl)
                n2925 = call "IR AOM freq to word.vi"("Frequency In (MHz)"=w3745) -> ("Frequency Word Out (double)"=w3742:dbl)
                n2926 = local write "Initializing"(FALSE ("Initializing")) -> ()
                n2927 = local write "Waiting"(TRUE ("Waiting")) -> ()
                n2928 = To Quad Integer(1:w3742) -> (0:w3741:i64)
                n2929 = xnode "Read/Write Control"("FPGA VI Reference In"=w3744, "error in"=w3743, "FPGA TTrig Thresh"=w3741) -> ("FPGA VI Reference Out"=w3738:T20, "error out"=w3737:errorcluster)
                n2930 = xnode "Read/Write Control"("FPGA VI Reference In"=w3738, "error in"=w3737, "FPGA Trap Trig"=TRUE) -> ()  [unwired: 2 out]
              }
            }
          }
        }
      }
    }
    n2931 = feedback-in #23(w3324) -> ()
    n2932 = feedback-in #24(w3321) -> ()
    n2933 = Split 1D Array(array=w3276, index=w3338) -> (first subarray=w3439:dbl[])  [unwired: 1 out]
    n2934 = feedback-in #25(w3439) -> ()
    n2935 = call-poly <vilib>:"Mean.vi"("X"=w3439) -> ("mean"=w3438:dbl)  [unwired: 1 out]
    "Bead Mean (nm)" <- w3438
    n2936 = Subtract(x=w3439, y=w3438) -> (x-y=w3437:dbl[])
    n2937 = Square(x=w3437) -> (x^2=w3436:dbl[])
    n2938 = call-poly <vilib>:"Mean.vi"("X"=w3436) -> ("mean"=w3435:dbl)  [unwired: 1 out]
    n2939 = Square Root(x=w3435) -> (sqrt(x)=w3434:dbl)
    n2940 = Multiply(x=10.0, y=w3434) -> (x*y=→"RMS (Ang)":dbl)
    n2941 = xnode ("Read/Write Control")("FPGA VI Reference In"=w3471, "error in"=w3470) -> ("FPGA VI Reference Out"=w3306:T20, "error out"=w3305:errorcluster, "AI2 Y Sum Set 1"=w3569:i16, "AI2 Y Sum Set 2"=w3568:i16, "AI1 X Set 1"=w3370:fxp<+/-,16,1>, "AI1 X Set 2"=w3369:fxp<+/-,16,1>, "Trap Pos FB Int Signal"=→"Trap Pos FB Int Signal":fxp<+/-,24,9>, "Trap Pos FB Int-Norm Signal"=→"Trap Pos FB Int-Norm Signal":fxp<+/-,16,1>, "Trap Pos FB Action"=w3363:i64, "Scanning"=→"AOD Scanning":bool, "Scan I"=→"AOD Scan I":u64, "Scanning MCL"=w3571:bool, "Scan I (MCL)"=→"MCL Scan I":u64, "Green FB Sum"=w3508:i16, "Trap Pos FB Action"=w3293:i64, "TTrig Fin Thresh"=w3289:i64, "Red FB Intensity"=w3270:i16, "Blue Intensity"=w3265:i16)
    "MCL Scanning" <- w3571
    "Trap Pos FB Action" <- w3363
    n2942 = Divide(x=w3270, y=3276.7) -> (x/y=w3269:dbl)
    "Red laser intensity (V)" <- w3269
    n2943 = Divide(x=w3265, y=3276.7) -> (x/y=w3264:dbl)
    "Blue laser intensity (V)" <- w3264
    n2944 = Divide(x=w3508, y=3276.7) -> (x/y=w3268:dbl)
    "Green laser intensity (V)" <- w3268
    n2945 = local read "FB Trig Integrate"() -> (w3287:u32)
    n2946 = Divide(x=w3293, y=w3287) -> (x/y=w3286:dbl)
    "TTrig Sig (Int)" <- w3286
    n2947 = Bundle(w3268, w3269, w3264) -> (→"Fluorescence laser intensities plot":cluster{dbl, dbl, dbl})  [unwired: 1 in]
    n2948 = Divide(x=w3289, y=w3287) -> (x/y=w3284:dbl)
    "TTrig Fin Thresh (Int)" <- w3284
    n2949 = local read "AOM X Cal (nm/MHz)"() -> (w3292:dbl)
    n2950 = local read "AI2 (V)"() -> (w3570:cluster{"Set 1":dbl, "Set 2":dbl})
    n2951 = Bundle By Name(cluster=w3570, "Set 1"=w3569, "Set 2"=w3568) -> (w3566:cluster{"Set 1":dbl, "Set 2":dbl})
    n2952 = Divide(x=w3363, y=327.67) -> (x/y=→"Action (%)":dbl)
    n2953 = local read "Trap X (AI1)"() -> (w3383:T10)
    n2954 = call "IR AOM word double to freq.vi"("Frequency Word In (double)"=w3284) -> ("Frequency Out (MHz)"=w3283:dbl)
    n2955 = call "IR AOM word double to freq.vi"("Frequency Word In (double)"=w3286) -> ("Frequency Out (MHz)"=w3285:dbl)
    n2956 = Divide(x=w3566, y=3276.7) -> (x/y=w3565:cluster{"Set 1":dbl, "Set 2":dbl})
    n2957 = Multiply(x=w3285, y=w3292) -> (x*y=w3291:dbl)
    "TTrig Sig (nm)" <- w3291
    n2958 = Multiply(x=w3283, y=w3292) -> (x*y=w3290:dbl)
    "TTrig Fin Thresh (nm)" <- w3290
    n2959 = local write "AI2 (V)"(w3565) -> ()
    n2960 = Bundle(cluster=w3383, "Trap 1"=w3370, "Trap 2"=w3369) -> (→"Trap X (AI1)":T10)
    n2961 = Bundle(w3291, w3290) -> (→"TTrig":cluster{dbl, dbl})  [unwired: 1 in]
    n2962 = flat-sequence "To save data" {
      tunnel: [w4655] -> w3589
      tunnel: [w4656] -> w3588
      tunnel: w3539 -> [w4649]
      tunnel: w3311 -> [w4653]
      tunnel: ["Save Calibration"] -> w3562
      tunnel: w3559 -> [w4652]
      tunnel: [w4645] -> w3558
      tunnel: [w4642] -> w3557
      tunnel: [w4639] -> w3556
      tunnel: w3538 -> [w4641]
      tunnel: w3453 -> [w4635]
      tunnel: [w4635] -> w3452
      tunnel: ["Start Saving"] -> w3422
      tunnel: [w4629] -> w3351
      tunnel: [w4628] -> w3350
      tunnel: w3589 -> [w4903]
      tunnel: w3588 -> [w4902]
      tunnel: w3352 -> [w4901]
      tunnel: w3562 -> [w4900]
      tunnel: w3558 -> [w4898]
      tunnel: w3557 -> [w4897]
      tunnel: w3556 -> [w4896]
      tunnel: w3431 -> [w4895]
      tunnel: w3463 -> [w4894]
      tunnel: w3452 -> [w4893]
      tunnel: w3422 -> [w4892]
      tunnel: w3420 -> [w4891]
      tunnel: w3248 -> [w4890]
      tunnel: w3351 -> [w4889]
      tunnel: w3350 -> [w4888]
      tunnel: w3349 -> [w4887]
      tunnel: w3272 -> [w4886]
      frame #0 {
        n2963 = Or(x="Save N Sets", y="Start Saving") -> (x .or. y?=w4636:bool)
        n2964 = To Double Precision Float(number=w4652) -> (double precision float=w4646:dbl)
        n2965 = Build Array(w4636, "Save Calibration", w4649, w4641) -> (w4651:bool[])
        n2966 = Compound Arithmetic op=OR("Save Calibration", w4649, w4636, w4641) -> (w4654:bool)
        n2967 = Boolean Array To Number(Boolean array=w4651) -> (number=w4648:u32)
        n2968 = feedback #27(FALSE ("Save APD Data\nwith Trap Data")) -> (w4630:bool)
        n2969 = feedback #28(refnum<k0> refnum) -> (w4657:refnum<file>)
        n2970 = feedback #29(refnum<k0> refnum) -> (w4632:refnum<file>)
        n2971 = feedback #30(FALSE ("Save APD Data\nwith Trap Data")) -> (w4640:bool)
        n2972 = feedback #31(refnum<k0> refnum) -> (w4643:refnum<file>)
        n2973 = feedback #32(0) -> (w4659:i32)
        n2974 = feedback #33() -> (w4647:u32)  [unwired: 1 out]
        n2975 = case shown="True" w4654 {
          tunnel: [w4666 1] -> w4655
          tunnel: w4659 -> [w4668 _]
          tunnel: [w4667 w4699] -> w4656
          tunnel: w4657 -> [w4667 _]
          tunnel: w4653 -> [_ w4717]
          tunnel: w4646 -> [_ w4715]
          tunnel: w4648 -> [_ w4718]
          tunnel: [w4665 w4698] -> w4645
          tunnel: w4647 -> [w4665 _]
          tunnel: [w4664 w4696] -> w4642
          tunnel: w4643 -> [w4664 _]
          tunnel: [w4663 w4695] -> w4639
          tunnel: w4640 -> [w4663 _]
          tunnel: "Start Saving" -> [_ w4693]
          tunnel: w4635 -> [_ w4692]
          tunnel: [w4662 w4684] -> w4628
          tunnel: w4632 -> [w4662 _]
          tunnel: [w4661 w4683] -> w4629
          tunnel: w4630 -> [w4661 _]
          frame False {
            n2976 = Increment(x=w4668) -> (x+1=w4666:i32)
          }
          frame True {
            w4689 = FALSE ("Start Saving")
            w4694 = 9.0  # File Version
            w4701 = FALSE ("prepend array or string size? (T)")
            w4700 = T28."big-endian, network order" ("byte order (0:big-endian, network order)")
            n2977 = local read "BD 1 Frequency 1 (MHz)"() -> (w4714:dbl)
            n2978 = local read "BD 2 Frequency 1 (MHz)"() -> (w4713:dbl)
            n2979 = local read "BD 1 Frequency 2 (MHz)"() -> (w4712:dbl)
            n2980 = local read "BD 2 Frequency 2 (MHz)"() -> (w4711:dbl)
            n2981 = local read "BD 1 Frequency 3 (MHz)"() -> (w4710:dbl)
            n2982 = local read "BD 2 Frequency 3 (MHz)"() -> (w4709:dbl)
            n2983 = Array Size(array=w4692) -> (size(s)=w4691:i32)
            n2984 = To Double Precision Float(number=w4691) -> (double precision float=w4690:dbl)
            n2985 = local write "Save Calibration"(w4689) -> ()
            n2986 = local write "Start Saving"(w4689) -> ()
            n2987 = Build Array("Save APD Data\nwith Trap Data", "Save Trap Pos. Data") -> (w4686:bool[])
            n2988 = Boolean Array To Number(Boolean array=w4686) -> (number=w4685:u32)
            n2989 = Build Array(w4714, w4713, w4712, w4711, w4710, w4709) -> (w4708:dbl[])
            n2990 = case shown="1, Default" w4718 {
              tunnel: w4717 -> [w4790 w4810 w4826 w4864]
              tunnel: w4690 -> [w4795 w4817 w4846 w4883]
              tunnel: w4715 -> [w4794 w4816 w4845 w4882]
              tunnel: [w4791 w4812 w4837 w4874] -> w4706
              tunnel: [w4782 "Cal sets to save" w4827 w4865] -> w4698
              tunnel: w4708 -> [w4792 w4813 w4839 w4876]
              tunnel: "Save APD Data\nwith Trap Data" -> [w4789 _ w4823 w4862]
              tunnel: [w4789 w4804 w4823 w4862] -> w4695
              tunnel: w4694 -> [w4785 w4805 w4821 w4860]
              tunnel: w4693 -> [w4784 _ _ _]
              tunnel: [w4775 w4804 w4820 w4850] -> w4683
              tunnel: "Save Trap Pos. Data" -> [w4775 _ w4820 w4850]
              tunnel: w4685 -> [w4774 _ w4819 w4849]
              frame 1, Default {
                # "timeseries"
                n2991 = case shown="True" "Profile" {
                  tunnel: [w4798 w4802] -> w4779
                  tunnel: [w4798 w4801] -> w4778
                  tunnel: [w4798 w4800] -> w4777
                  tunnel: [w4798 w4799] -> w4776
                  frame False {
                    w4798 = 0.0 ("f")
                  }
                  frame True {
                    n2992 = local read "Current Position"() -> (w4803:cluster{dbl, dbl, dbl})
                    n2993 = local read "Y change (mm)"() -> (w4799:dbl)
                    n2994 = Unbundle(w4803) -> (w4802:dbl, w4801:dbl, w4800:dbl)
                  }
                }
                n2995 = local read "Save ave N"() -> (w4797:dbl)
                n2996 = Multiply(x=w4797, y=w4790) -> (x*y=w4796:dbl)
                n2997 = To Double Precision Float(number=w4774) -> (double precision float=w4788:dbl)
                n2998 = Build Array(w4785, w4790, w4796, w4795, w4794, 0.0 ("f")) -> (w4793:dbl[])
                n2999 = Build Array(w4788, w4779, w4778, w4777, w4776) -> (w4786:dbl[])
                n3000 = Select(t=u32 4000000000, s=w4784, f="N sets to save") -> (s? t:f=w4782:u32)
                n3001 = Build Array (concatenate)(w4793, w4792, w4786) -> (w4791:dbl[])
              }
              frame 2 {
                w4807 = 0.0 ("f")
                w4804 = FALSE ("Save APD Data\nwith Trap Data")
                # "calibration"
                n3002 = Boolean To (0,1)(Boolean=w4804) -> (0, 1=w4809:i16)
                n3003 = To Double Precision Float(number=w4809) -> (double precision float=w4808:dbl)
                n3004 = Build Array(w4808, w4807, w4807, w4807, w4807) -> (w4806:dbl[])
                n3005 = Build Array(w4805, w4810, w4810, w4817, w4816, 1.0 ("t")) -> (w4814:dbl[])